vi "rydberg_trigger_snap.vi"() -> ()   [LabVIEW 2013]
uses:
  instrumentvi_Neutral/cameratrigger/related_vi/check_pixelfly_status.vi
  <vilib>/Utility/file.llb/Read From Spreadsheet File (DBL).vi
  <vilib>/Utility/file.llb/Write To Spreadsheet File (DBL).vi
panel:
  in  "Case Constant\n(See Context Help) 2":bool
  in  "Case Constant\n(See Context Help)":bool
  out "iteration#":i32=25
  in  "Turn channels ON/OFF\n(works in real time)":bool[](array[boolean])=[TRUE, TRUE, FALSE, FALSE, FALSE, FALSE, FALSE, FALSE, FALSE, FALSE, FALSE, FALSE, FALSE, FALSE, FALSE, FALSE]
  in  "Save data every nth iteration":dbl=25.0
  out "Analog Input \nVoltage Monitor":T1(graph)={"data[0]"=-0.7588496337314492, "data[1]"=-0.07985869959699164, "data[2]"=0.0, "data[3]"=0.0, "data[4]"=0.0, "data[5]"=0.0, "data[6]"=0.0, "data[7]"=0.0, "data[8]"=0.0, "data[9]"=0.0, "data[10]"=0.0, "data[11]"=0.0, "data[12]"=0.0, "data[13]"=0.0, "data[14]"=0.0, "data[15]"=0.0}
  in  "Tab Control":enum32{"Controls", "Images", "Status"}(tab)=enum."Images"
  in  "Voltage Log File Path":path=path "C:/data/Voltage Log Files/voltagelog011708.txt"
  in  "Monitor voltages?":bool
  in  "Voltage\nMonitor\nControl":u16(ring)=1 caption="Voltage Monitor Control" items=["Off", "Each imaging cycle", "Verdi temp mon"]
  out "DoubleShutter?":bool=TRUE
  in  "File Path for Electronic Background Image":path=path "C:/data/tempfiles/junkeback.dat"
  in  "File Path for Atoms":path=path "C:/data/tempfiles/junkatoms.dat"
  in  "File Path for Background":path=path "C:/data/tempfiles/junkback.dat"
  in  "Timeout (min 100 ms)":u32=1000
  in  "Max Iteration (timeout)":i32=51
  in  "Camera background with no image beam.\nIt will be subtracted before the log is taken":i16 min=0
  in  "Software Bin Size":i32=2
  in  "Software Binning?":bool=TRUE
  in  "Subtract Electronic BG?":bool
  in  "Cut Image?":bool=TRUE
  in  "ROI Parameters":T2={"Col Start"=250, "Col Stop"=550, "Row Start"=1025, "Row stop"=1225} {"Row stop" min=1 max=1280; "Row Start" min=1 max=1280; "Col Stop" min=1 max=1024; "Col Start" min=1 max=1024}
  in  "Coil Current (amps)":dbl=34.0 format="%.2f"
  in  "Natural Linewidth of Transition (in MHz)":dbl=32.0
  in  "Image Beam Detuning (MHz)":dbl format="%.2f"
  in  "Image Beam Wavelength (m)":dbl=4.61e-07
  in  "Number for Scale":dbl=5.0
  in  "Number of Pixels to Smooth":dbl=1.0
  in  "Cut Borders":dbl
  in  "Limit":dbl=5.0
  in  "Sample Interleave":dbl=1.0 min=1.0
  in  "Pixel Size (m)":dbl=6e-06
  in  "Scale Base Level?":bool
  in  "1D Fit On?":bool=TRUE
  in  "2D Fit On?":bool=TRUE
  out "boardid (indicator)":i32
  in  "Gain":i32(ring) items=["Low (X1)", "High (X2)"]
  in  "Exp Time: This sets first image exposure and start of image readout. Make sure you account for this time.":i32=1000 min=1 max=10000
  in  "V Bin":i32(ring) items=["1", "2"]
  in  "H Bin":i32(ring) items=["1", "2"]
  in  "Exp Level":i32=1 min=0 max=255 step=1
  in  "Trigger":bool=TRUE
  in  "Exposure Mode":u16(ring)=1 items=["Asynch shutter", "Double shot", "Video mode", "Auto exposure"]
  out "?":ext format="%.2f"
  in  "?":i32=35
  in  "?":i32=87
  out "PixelFly Status":bool
  out "Atoms - Background at Analysis Size":dbl[][](graph)
  out "image -  bg sum of ROI from back":dbl(graph)=-492168.0
  out "Last 40 numbers":dbl(graph)
  out "Atoms Image":dbl[][](graph)
  out "Atoms - Background":dbl[][](graph)
  out "parameters from \npeak absorption":T3={"alpha"=1.0152277070063695e-13, "peakdensity"=4.819850374584978e+17, "alphadenssigzsqrt2pi"=2.914507, "number"=142895.21998245403} {"number" format="%.3e"; "alphadenssigzsqrt2pi" format="%.3e"; "peakdensity" format="%.3e"; "alpha" format="%.3e"}
  out "Image Size for Analysis":i32[](array[numeric])=[150, 100]
  out "peak OD":dbl format="%#_4g"
  in  "# Images to Sum":i32=1
  in  "Continuous Scan?\n(No Images Saved)":bool=TRUE
  in  "Autoscale\nRoutine On?":bool
  in  "Analyze \nImages?":bool=TRUE
  out "# of Current Image":i32=1
  in  "Camera Function":i32(ring)=2 items=["Camera Initialize", "Acquire", "Shutdown"]
  in  "Stop Continuous Scan?":bool
  out "2D Fit Chi-squared":dbl format="%#_3g"
  out "Num Atoms - OD Integral":dbl format="%#_4g"
  out "Num Atoms - Peak OD":dbl format="%#_4g"
  out "Y 1D Fit Values":T4={"Amplitude"=17.90491094333259, "y0"=0.0006453741239587313, "rmswidthy"=3.333942391455422e-05, "offsety"=-3.142553421752575, "Number Y"=176863.40216585185} {"Number Y" format="%.2e"; "offsety" format="%.2e"; "rmswidthy" format="%.2e"; "y0" format="%.2e"; "Amplitude" format="%.2e"}
  out "X 1D Fit Values":T5={"Amplitude"=24.47847782439825, "x0"=0.0009429207504454069, "rmswidthx"=2.376173376668835e-05, "offsetx"=-2.0737454877905925, "Number X"=172333.71575846447} {"Number X" format="%.2e"; "offsetx" format="%.2e"; "rmswidthx" format="%.2e"; "x0" format="%.2e"; "Amplitude" format="%.2e"}
  out "2-D Fit Parameters":T6
  out "Avg Back":ext=1449.7175567626953 format="%.2e"
  out "Avg Atoms-Back":ext=-7.78399887084961 format="%.2e"
  out "Avg Atoms":ext=1441.9335578918458 format="%.2e"
  out "Opticaldepthimagesingle (ln(atoms)-ln(back))(-1)":dbl[][](graph)
  out "Smoothed OD - Fit OD":dbl[][](graph)
  out "Uncut Image - Doubleshot":dbl[][](graph)
  out "Y density distribution: log(sum_x atoms) -log(sum_x backgnd)":cluster{dbl[], dbl[]}[](graph)=[{[0.0, 1.2e-05, 2.4e-05, 3.6e-05, 4.8e-05, 6e-05, 7.2e-05, 8.400000000000001e-05, 9.6e-05, 0.000108, 0.00012, 0.000132, 0.000144, 0.000156, 0.00016800000000000002, 0.00018, 0.000192, 0.000204, 0.000216, 0.000228, 0.00024, 0.000252, 0.000264, 0.000276, 0.000288, 0.00030000000000000003, 0.000312, 0.000324, 0.00033600000000000004, 0.000348, 0.00036, 0.000372, 0.000384, 0.00039600000000000003, 0.000408, 0.00042, 0.000432, 0.000444, 0.000456, 0.000468, 0.00048, 0.000492, 0.000504, 0.000516, 0.000528, 0.00054, 0.000552, 0.000564, 0.000576, 0.000588, 0.0006000000000000001, 0.000612, 0.000624, 0.0006360000000000001, 0.000648, 0.00066, 0.0006720000000000001, 0.000684, 0.000696, 0.000708, 0.00072, 0.000732, 0.000744, 0.000756, 0.000768, 0.00078, 0.0007920000000000001, 0.000804, 0.000816, 0.0008280000000000001, 0.00084, 0.000852, 0.000864, 0.000876, 0.000888, 0.0009, 0.000912, 0.000924, 0.000936, 0.0009480000000000001, 0.00096, 0.000972, 0.000984, 0.000996, 0.001008, 0.00102, 0.001032, 0.001044, 0.001056, 0.001068, 0.00108, 0.001092, 0.001104, 0.001116, 0.001128, 0.00114, 0.001152, 0.001164, 0.001176, 0.001188], [-3.3686591448665695, -3.3593416907117444, -2.501141797799619, -3.137266718233832, -3.587719306130566, -2.6390745848241295, -3.6966092446853054, -2.6808187998242374, -3.0319112156403207, -2.7363781603955886, -3.363138854673707, -2.731002614818408, -3.3935197594450983, -3.0493035465378853, -3.2941032756557433, -3.092209549305835, -3.0943983454935733, -3.2393686037710268, -2.730035543135955, -3.287849371356515, -2.5686023814239434, -3.1088703551167782, -2.856653458062283, -3.240447915604136, -3.4894394818825276, -2.9961131164766357, -4.104169957056229, -2.8255474959485127, -3.8878748767015168, -3.0775415698653887, -3.7197529539632797, -3.3776657935209187, -3.8047169273982036, -3.4536401406066943, -3.3930728929356064, -3.1293918380520154, -3.433923718918095, -2.8153587940721536, -3.6029531308467995, -2.4989306176071295, -3.483829652183431, -2.9711985693618317, -3.697510544320039, -3.1132099718149675, -3.803881645787669, -3.6495652439025434, -3.6485837854809233, -3.185441611433589, -1.652208255575033, 0.03140941165247568, 4.4569342541294645, 8.56173788023807, 12.377374823114451, 13.49419715605518, 13.361094012986996, 13.08877719779457, 10.635138116352437, 6.592571400876977, 2.8347368854219894, -0.6335944505865427, -2.5137500326873123, -3.043489857024497, -2.68801842384687, -3.0676047259767074, -2.9163649829733913, -3.168337622954141, -2.7690334242099652, -3.322776293644665, -3.119521162448791, -3.04783132514558, -2.619550840819329, -3.2013707187938962, -2.419650797146687, -2.902692626093767, -3.0917951318126597, -2.8856469922691304, -3.523759843666312, -3.0084041621928463, -3.646833134218241, -3.1529925921761333, -3.371597483779624, -3.5211395371050003, -3.153552371623391, -3.4981555573237983, -3.7751962171532796, -2.992402620435996, -3.2399196976318763, -2.831696410884433, -2.7750651929482046, -2.8873123361618127, -2.360377205045097, -2.399998629312904, -2.590436576132106, -2.2120804438281993, -2.5532249988086733, -2.7154620505466482, -2.369902307173561, -3.201516908291751, -2.571788439326383, -2.629373703639885]}, {[0.0, 1.2e-05, 2.4e-05, 3.6e-05, 4.8e-05, 6e-05, 7.2e-05, 8.400000000000001e-05, 9.6e-05, 0.000108, 0.00012, 0.000132, 0.000144, 0.000156, 0.00016800000000000002, 0.00018, 0.000192, 0.000204, 0.000216, 0.000228, 0.00024, 0.000252, 0.000264, 0.000276, 0.000288, 0.00030000000000000003, 0.000312, 0.000324, 0.00033600000000000004, 0.000348, 0.00036, 0.000372, 0.000384, 0.00039600000000000003, 0.000408, 0.00042, 0.000432, 0.000444, 0.000456, 0.000468, 0.00048, 0.000492, 0.000504, 0.000516, 0.000528, 0.00054, 0.000552, 0.000564, 0.000576, 0.000588, 0.0006000000000000001, 0.000612, 0.000624, 0.0006360000000000001, 0.000648, 0.00066, 0.0006720000000000001, 0.000684, 0.000696, 0.000708, 0.00072, 0.000732, 0.000744, 0.000756, 0.000768, 0.00078, 0.0007920000000000001, 0.000804, 0.000816, 0.0008280000000000001, 0.00084, 0.000852, 0.000864, 0.000876, 0.000888, 0.0009, 0.000912, 0.000924, 0.000936, 0.0009480000000000001, 0.00096, 0.000972, 0.000984, 0.000996, 0.001008, 0.00102, 0.001032, 0.001044, 0.001056, 0.001068, 0.00108, 0.001092, 0.001104, 0.001116, 0.001128, 0.00114, 0.001152, 0.001164, 0.001176, 0.001188], [-3.142553421752575, -3.142553421752575, -3.142553421752575, -3.142553421752575, -3.142553421752575, -3.142553421752575, -3.142553421752575, -3.142553421752575, -3.142553421752575, -3.142553421752575, -3.142553421752575, -3.142553421752575, -3.142553421752575, -3.142553421752575, -3.142553421752575, -3.142553421752575, -3.142553421752575, -3.142553421752575, -3.142553421752575, -3.142553421752575, -3.142553421752575, -3.142553421752575, -3.142553421752575, -3.142553421752575, -3.142553421752575, -3.142553421752575, -3.142553421752575, -3.142553421752575, -3.142553421752575, -3.142553421752575, -3.142553421752573, -3.14255342175253, -3.1425534217517685, -3.1425534217398705, -3.1425534215767574, -3.142553419615115, -3.142553398924452, -3.142553207572838, -3.1425516564361646, -3.1425406396371858, -3.1424721164431455, -3.1420990921048606, -3.1403231424865408, -3.1329354518498045, -3.106116340729864, -3.021287229549591, -2.788007984145684, -2.231927393950265, -1.0878733189191243, 0.9301648516208109, 3.9493125759985808, 7.706020947338827, 11.43621434642004, 14.068401345797076, 14.706907582526853, 13.11971957540532, 9.873322089660576, 6.009141262246697, 2.510273096557114, -0.0751860764137236, -1.680369782741332, -2.530239620690055, -2.917294410160682, -3.0697542735255157, -3.1218850426129303, -3.137398494519852, -3.1414239518658547, -3.1423360201347044, -3.1425166607891493, -3.1425479610692, -3.1425527091570276, -3.142553340061387, -3.1425534135255404, -3.142553421024716, -3.1425534216960047, -3.1425534217487128, -3.142553421752343, -3.142553421752563, -3.1425534217525746, -3.142553421752575, -3.142553421752575, -3.142553421752575, -3.142553421752575, -3.142553421752575, -3.142553421752575, -3.142553421752575, -3.142553421752575, -3.142553421752575, -3.142553421752575, -3.142553421752575, -3.142553421752575, -3.142553421752575, -3.142553421752575, -3.142553421752575, -3.142553421752575, -3.142553421752575, -3.142553421752575, -3.142553421752575, -3.142553421752575, -3.142553421752575]}]
  out "Intensity v/s X":cluster{dbl[], dbl[]}[](graph)=[{[0.0, 1.2e-05, 2.4e-05, 3.6e-05, 4.8e-05, 6e-05, 7.2e-05, 8.400000000000001e-05, 9.6e-05, 0.000108, 0.00012, 0.000132, 0.000144, 0.000156, 0.00016800000000000002, 0.00018, 0.000192, 0.000204, 0.000216, 0.000228, 0.00024, 0.000252, 0.000264, 0.000276, 0.000288, 0.00030000000000000003, 0.000312, 0.000324, 0.00033600000000000004, 0.000348, 0.00036, 0.000372, 0.000384, 0.00039600000000000003, 0.000408, 0.00042, 0.000432, 0.000444, 0.000456, 0.000468, 0.00048, 0.000492, 0.000504, 0.000516, 0.000528, 0.00054, 0.000552, 0.000564, 0.000576, 0.000588, 0.0006000000000000001, 0.000612, 0.000624, 0.0006360000000000001, 0.000648, 0.00066, 0.0006720000000000001, 0.000684, 0.000696, 0.000708, 0.00072, 0.000732, 0.000744, 0.000756, 0.000768, 0.00078, 0.0007920000000000001, 0.000804, 0.000816, 0.0008280000000000001, 0.00084, 0.000852, 0.000864, 0.000876, 0.000888, 0.0009, 0.000912, 0.000924, 0.000936, 0.0009480000000000001, 0.00096, 0.000972, 0.000984, 0.000996, 0.001008, 0.00102, 0.001032, 0.001044, 0.001056, 0.001068, 0.00108, 0.001092, 0.001104, 0.001116, 0.001128, 0.00114, 0.001152, 0.001164, 0.001176, 0.001188, 0.0012000000000000001, 0.001212, 0.001224, 0.0012360000000000001, 0.001248, 0.00126, 0.0012720000000000001, 0.001284, 0.001296, 0.0013080000000000001, 0.00132, 0.001332, 0.0013440000000000001, 0.001356, 0.001368, 0.00138, 0.001392, 0.001404, 0.001416, 0.001428, 0.00144, 0.001452, 0.001464, 0.001476, 0.001488, 0.0015, 0.001512, 0.001524, 0.001536, 0.0015480000000000001, 0.00156, 0.001572, 0.0015840000000000001, 0.001596, 0.001608, 0.0016200000000000001, 0.001632, 0.001644, 0.0016560000000000001, 0.001668, 0.00168, 0.0016920000000000001, 0.001704, 0.001716, 0.001728, 0.00174, 0.001752, 0.001764, 0.001776, 0.001788], [-2.8183440721355737, -2.401522563761773, -2.5237601060707675, -2.500570399573121, -2.506086929574394, -2.3798757992705077, -2.491986345524083, -2.488259685244998, -2.5954764602082605, -2.6088044268195745, -2.565883062250009, -2.640123527845276, -2.5258645679890606, -2.542319425147525, -2.3663141562295777, -2.491158449081013, -2.4827761290987382, -2.5697565230360624, -2.675555471134544, -2.4526500510070264, -2.587401679302161, -2.7170704998887913, -2.5610989943488676, -2.5911334487145723, -2.5002374964478804, -2.4884694389456854, -2.5394904176372393, -2.5500867554972046, -2.378216817131488, -2.5395407567208395, -2.046418844121149, -2.1733857420010736, -2.669858427788313, -2.2304504062857404, -2.586975439308276, -2.4213636413369386, -2.3929041134997533, -2.488418399790703, -2.2930625821045396, -2.6069475160815045, -2.511643300766991, -2.273400532704045, -2.2899489155247466, -2.528198542008795, -2.357612131615724, -2.3432177912642373, -2.3168511287027513, -2.420032372065748, -2.395414080287992, -2.3757390661600084, -2.4716707833126748, -2.2185297028257764, -2.2814791274250865, -2.118623996360043, -2.0182357551965424, -2.432618062946176, -2.230506420081042, -2.146155705062938, -2.3472190640306962, -2.3712543536693147, -2.1875881775472408, -2.1952908358917966, -2.053287952368919, -1.8502300747721847, -1.9848473505809352, -1.9942680470508094, -2.0174521250165753, -2.0969782433525097, -1.8219170436304921, -1.6672326334789886, -1.4869217102946095, -0.9996339197143698, -0.8098748137616667, -0.35967428953222225, -0.650012388682967, 1.7919178156766975, 7.743635801250548, 16.428591835436464, 22.663725551287143, 20.240706904645776, 16.936256193013378, 9.701135845766885, 4.174916332451744, -0.2899352730639748, -1.661331740025389, -1.5080821335172914, -1.9026215949503467, -2.049002401491748, -1.9706402437938095, -2.0311585837459916, -2.077597516112178, -1.930667645093763, -2.1086022731634557, -1.7650030212055299, -1.917311464733416, -1.8111299981898128, -2.075459160990931, -2.2079166808241553, -1.8235763980834463, -1.898222513860219, -1.9621602868612626, -2.0017564868267073, -1.7095965014406147, -2.0323342222595784, -1.6211606697328307, -1.839833902685882, -1.9658503587635323, -1.9776012347161895, -1.887885369120113, -1.9468724100556756, -1.6351243930344026, -1.6613815392586275, -1.6219275265368651, -1.7589024364108354, -1.6045421848466503, -1.8391976965150434, -1.6203149700231734, -1.7969550536250836, -1.5575704192364128, -1.8258635266791998, -1.9097093493073771, -1.8343058761104203, -1.660627277068329, -1.945166122309729, -1.5463727138680952, -1.569489672727741, -1.6225878206881816, -1.7324496472705277, -1.631544148883222, -1.8227215123275755, -1.8797703918872912, -1.8647363562896544, -1.576905869043685, -1.970412155507347, -2.0096411488008243, -1.7813961287674829, -1.8489792019571496, -1.7513334844093151, -1.6826445124467, -1.8905109948545942, -1.7110939804845202, -1.7394070082149256, -1.599355827269278, -1.686777376633131, -1.4884369858077662, -1.653664890583741, -1.8092625318996625, -1.4833808568982931, -1.6619157448002397, -1.371210367738854]}, {[0.0, 1.2e-05, 2.4e-05, 3.6e-05, 4.8e-05, 6e-05, 7.2e-05, 8.400000000000001e-05, 9.6e-05, 0.000108, 0.00012, 0.000132, 0.000144, 0.000156, 0.00016800000000000002, 0.00018, 0.000192, 0.000204, 0.000216, 0.000228, 0.00024, 0.000252, 0.000264, 0.000276, 0.000288, 0.00030000000000000003, 0.000312, 0.000324, 0.00033600000000000004, 0.000348, 0.00036, 0.000372, 0.000384, 0.00039600000000000003, 0.000408, 0.00042, 0.000432, 0.000444, 0.000456, 0.000468, 0.00048, 0.000492, 0.000504, 0.000516, 0.000528, 0.00054, 0.000552, 0.000564, 0.000576, 0.000588, 0.0006000000000000001, 0.000612, 0.000624, 0.0006360000000000001, 0.000648, 0.00066, 0.0006720000000000001, 0.000684, 0.000696, 0.000708, 0.00072, 0.000732, 0.000744, 0.000756, 0.000768, 0.00078, 0.0007920000000000001, 0.000804, 0.000816, 0.0008280000000000001, 0.00084, 0.000852, 0.000864, 0.000876, 0.000888, 0.0009, 0.000912, 0.000924, 0.000936, 0.0009480000000000001, 0.00096, 0.000972, 0.000984, 0.000996, 0.001008, 0.00102, 0.001032, 0.001044, 0.001056, 0.001068, 0.00108, 0.001092, 0.001104, 0.001116, 0.001128, 0.00114, 0.001152, 0.001164, 0.001176, 0.001188, 0.0012000000000000001, 0.001212, 0.001224, 0.0012360000000000001, 0.001248, 0.00126, 0.0012720000000000001, 0.001284, 0.001296, 0.0013080000000000001, 0.00132, 0.001332, 0.0013440000000000001, 0.001356, 0.001368, 0.00138, 0.001392, 0.001404, 0.001416, 0.001428, 0.00144, 0.001452, 0.001464, 0.001476, 0.001488, 0.0015, 0.001512, 0.001524, 0.001536, 0.0015480000000000001, 0.00156, 0.001572, 0.0015840000000000001, 0.001596, 0.001608, 0.0016200000000000001, 0.001632, 0.001644, 0.0016560000000000001, 0.001668, 0.00168, 0.0016920000000000001, 0.001704, 0.001716, 0.001728, 0.00174, 0.001752, 0.001764, 0.001776, 0.001788], [-2.0737454877905925, -2.0737454877905925, -2.0737454877905925, -2.0737454877905925, -2.0737454877905925, -2.0737454877905925, -2.0737454877905925, -2.0737454877905925, -2.0737454877905925, -2.0737454877905925, -2.0737454877905925, -2.0737454877905925, -2.0737454877905925, -2.0737454877905925, -2.0737454877905925, -2.0737454877905925, -2.0737454877905925, -2.0737454877905925, -2.0737454877905925, -2.0737454877905925, -2.0737454877905925, -2.0737454877905925, -2.0737454877905925, -2.0737454877905925, -2.0737454877905925, -2.0737454877905925, -2.0737454877905925, -2.0737454877905925, -2.0737454877905925, -2.0737454877905925, -2.0737454877905925, -2.0737454877905925, -2.0737454877905925, -2.0737454877905925, -2.0737454877905925, -2.0737454877905925, -2.0737454877905925, -2.0737454877905925, -2.0737454877905925, -2.0737454877905925, -2.0737454877905925, -2.0737454877905925, -2.0737454877905925, -2.0737454877905925, -2.0737454877905925, -2.0737454877905925, -2.0737454877905925, -2.0737454877905925, -2.0737454877905925, -2.0737454877905925, -2.0737454877905925, -2.0737454877905925, -2.0737454877905925, -2.0737454877905925, -2.0737454877905925, -2.0737454877905925, -2.0737454877905925, -2.0737454877905925, -2.0737454877905925, -2.0737454877905925, -2.0737454877905925, -2.0737454877905925, -2.073745487790578, -2.073745487789698, -2.073745487748773, -2.0737454862751323, -2.073745445235809, -2.0737445618346193, -2.073729875366191, -2.073541507399717, -2.0716803713160936, -2.0575446026371003, -1.9752602822028478, -1.6098273966897678, -0.3803839855887031, 2.715820000636734, 8.423627049166667, 15.754276644617699, 21.388186935825832, 21.85183342897553, 16.8322343699678, 9.50266684232387, 3.41896670995723, -0.05427383695049559, -1.4984026137046382, -1.9467308492977926, -2.052017531704562, -2.0708652918518737, -2.0734496434587752, -2.0737219404138356, -2.0737440354787706, -2.073745418381675, -2.073745485220145, -2.0737454877168293, -2.073745487788952, -2.073745487790564, -2.073745487790592, -2.0737454877905925, -2.0737454877905925, -2.0737454877905925, -2.0737454877905925, -2.0737454877905925, -2.0737454877905925, -2.0737454877905925, -2.0737454877905925, -2.0737454877905925, -2.0737454877905925, -2.0737454877905925, -2.0737454877905925, -2.0737454877905925, -2.0737454877905925, -2.0737454877905925, -2.0737454877905925, -2.0737454877905925, -2.0737454877905925, -2.0737454877905925, -2.0737454877905925, -2.0737454877905925, -2.0737454877905925, -2.0737454877905925, -2.0737454877905925, -2.0737454877905925, -2.0737454877905925, -2.0737454877905925, -2.0737454877905925, -2.0737454877905925, -2.0737454877905925, -2.0737454877905925, -2.0737454877905925, -2.0737454877905925, -2.0737454877905925, -2.0737454877905925, -2.0737454877905925, -2.0737454877905925, -2.0737454877905925, -2.0737454877905925, -2.0737454877905925, -2.0737454877905925, -2.0737454877905925, -2.0737454877905925, -2.0737454877905925, -2.0737454877905925, -2.0737454877905925, -2.0737454877905925, -2.0737454877905925, -2.0737454877905925, -2.0737454877905925, -2.0737454877905925, -2.0737454877905925, -2.0737454877905925]}] caption="X Density Distribution: log(sum_y atoms) -log(sum_y backgnd)"
  out "Background Image":dbl[][](graph)
  out "Strip Chart\nerror out":errorcluster
  in  "Strip Chart\nerror in":errorcluster
  out "Strip chart counter":dbl
  out "initialized array":u8[][](array[numeric])
  in  "error in":errorcluster
  out "error out":errorcluster={"status"=TRUE, "code"=-131, "source"="Remove buffer from list.vi: Picture buffer already in use"} caption="Camera Error Out 1"
  out "error out 2":errorcluster={"status"=FALSE, "code"=0, "source"="Start camera.vi: No error - function call successful"} caption="Camera Error Out 2"
  out "Camera Error Out 3":errorcluster={"status"=FALSE, "code"=0, "source"="Get buffer status.vi: No error - function call successful"}
  out "V bin 2":i32(ring) items=["1", "2"]
  out "H bin 2":i32(ring) items=["1", "2"]
  out "Buffer number":i32=1
  out "Size":i32=5242880
  out "Buffer address":i32=241958912
  out "Camera Board Parameters":T7={"Type"=65, "Number"=1, "Initialized"=TRUE, "Running"=TRUE, "Lost head"=FALSE, "CCD X size"=1280, "CCD Y size"=1024, "Mode"=32, "Exposure time"=1000, "Exposure level"=1, "Horizontal bin"=0, "Vertical bin"=0, "Reg W"=FALSE, "Gain"=0, "Pixel depth"=12, "Bit Shift"=0, "Offset"=0, "Last exposure"=1000, "Double "=TRUE, "Light meter"=FALSE, "Color"=FALSE, "Open count"=2295301936, "Active buffer"=TRUE, "Next Buffer"=TRUE} {"Vertical bin" items=["1", "2"]; "Horizontal bin" items=["1", "2"]}
  out "Camera Buffer status":T8={"Write"=FALSE, "Write done"=TRUE, "Queued"=FALSE, "Cancelled"=FALSE, "Select"=FALSE, "Select done"=FALSE, "Burst"=FALSE, "Size"=FALSE, "Event"=FALSE, "Timeout"=FALSE, "Open"=0, "Map"=4372, "Exposure"=[1000], "Offset"=[0], "Size"=[5242880], "Transfer"=[0], "Total Size"=392691712}
  in  "offset":i32
  out "Output ClusterY\n(arb fit)":T9={"amplitudey"=0.008995711509471623, "temperaturey"=0.002709094402736608, "alphay"=0.0011778671316246122, "offsety"=-0.0002344292151486787, "numbery"=771798750.645837, "peakdensityy"=4696134676573208.0, "centery"=0.004923587672892697} {"centery" format="%.2e"; "peakdensityy" format="%.2e"; "numbery" format="%.2e"; "offsety" format="%.2e"; "alphay" format="%.2e"; "temperaturey" format="%.2e"; "amplitudey" format="%.2e"}
  out "Output Cluster X\n(arb fit)":T10={"amplitudex"=0.0047697219685124154, "temperaturex"=0.0023439442598952344, "alphax"=0.0010191061999544498, "offsetx"=8.440276213188199e-05, "numberx"=708132868.1536969, "peakdensityx"=6652452808873044.0, "centerx"=0.0037182148271134325} {"centerx" format="%.2e"; "peakdensityx" format="%.2e"; "numberx" format="%.2e"; "offsetx" format="%.2e"; "alphax" format="%.2e"; "temperaturex" format="%.2e"; "amplitudex" format="%.2e"}
  out "Y side(by arbfit)":cluster{cluster{dbl, dbl}[]}[](graph)=[{[{0.0, -9.666143798828125e-05}, {4.63e-05, 4.321251220703125e-05}, {9.26e-05, -0.00016961046142578126}, {0.00013890000000000002, -0.0001606823974609375}, {0.0001852, -3.920782470703125e-05}, {0.0002315, -0.000111915087890625}, {0.00027780000000000003, -0.00018772257080078126}, {0.0003241, -0.00014607723388671877}, {0.0003704, 3.730218505859375e-05}, {0.0004167, -0.000120493310546875}, {0.000463, -2.0831201171875e-05}, {0.0005093, 8.1265576171875e-05}, {0.0005556000000000001, -4.6981127929687503e-05}, {0.0006019, 2.730753173828125e-05}, {0.0006482, 0.0001042299560546875}, {0.0006945, 8.897061767578125e-05}, {0.0007408, -0.0001128991943359375}, {0.0007871, -3.39658935546875e-05}, {0.0008334, 0.00021708648681640627}, {0.0008797, 1.521951904296875e-05}, {0.000926, -8.81429443359375e-05}, {0.0009723, 0.00017849017333984376}, {0.0010186, 0.00016118013916015624}, {0.0010649, 4.3130029296875e-05}, {0.0011112000000000001, 0.000101584814453125}, {0.0011575000000000001, 0.0001667121826171875}, {0.0012038, 0.0001330364013671875}, {0.0012501, 1.435771484375e-05}, {0.0012964, 0.00013017509765625}, {0.0013427, 0.0001979874267578125}, {0.001389, 0.0001995517578125}, {0.0014353, 5.386134033203125e-05}, {0.0014816, 0.00013825557861328125}, {0.0015279, 0.00037487060546875003}, {0.0015742, 0.0001915253173828125}, {0.0016205, 0.000173282373046875}, {0.0016668, 0.00030387272949218753}, {0.0017131, 0.0005522344604492188}, {0.0017594, 0.0003743757080078125}, {0.0018057, 0.000244183544921875}, {0.001852, 0.0004390764404296875}, {0.0018983000000000001, 0.0004536360961914063}, {0.0019446, 0.00044938680419921874}, {0.0019909, 0.00031516435546875}, {0.0020372, 0.0003973002685546875}, {0.0020835, 0.000558414990234375}, {0.0021298, 0.0005315966674804687}, {0.0021761, 0.00047105989990234374}, {0.0022224000000000002, 0.0006024039794921875}, {0.0022687000000000002, 0.0006190456176757812}, {0.0023150000000000002, 0.0006605089233398438}, {0.0023613, 0.0006151063476562501}, {0.0024076, 0.0007049785888671875}, {0.0024539, 0.0008554387939453125}, {0.0025002, 0.000755099755859375}, {0.0025465, 0.0008008635498046875}, {0.0025928, 0.0007846542358398437}, {0.0026391, 0.00092633427734375}, {0.0026854, 0.0009349409423828125}, {0.0027317, 0.0009390679321289063}, {0.002778, 0.0009715178466796875}, {0.0028243, 0.0009944736938476563}, {0.0028706, 0.001180484033203125}, {0.0029169, 0.0010933195068359375}, {0.0029632, 0.0010906231689453126}, {0.0030095, 0.0010906317016601563}, {0.0030558, 0.0013240981567382813}, {0.0031021, 0.0014536930297851564}, {0.0031484, 0.001447785546875}, {0.0031947, 0.0013987793212890626}, {0.003241, 0.0015179443725585938}, {0.0032873, 0.0015591374755859375}, {0.0033336, 0.0016731800537109376}, {0.0033799, 0.0016079417602539064}, {0.0034262, 0.0015991075561523438}, {0.0034725, 0.0018513971801757813}, {0.0035188, 0.0018405805419921875}, {0.0035651, 0.0018605926025390626}, {0.0036114, 0.001904240283203125}, {0.0036577, 0.0018782012817382813}, {0.003704, 0.0019519751342773437}, {0.0037503000000000002, 0.0020929782470703127}, {0.0037966000000000002, 0.002198195153808594}, {0.0038429000000000002, 0.0021514216552734377}, {0.0038892, 0.0020961069091796876}, {0.0039355, 0.002265489831542969}, {0.0039818, 0.0023468663330078127}, {0.0040281, 0.002427193310546875}, {0.0040744, 0.0024689637939453125}, {0.0041207, 0.0024438804565429686}, {0.004167, 0.0024601580322265626}, {0.0042133, 0.002636688525390625}, {0.0042596, 0.002699147998046875}, {0.0043059, 0.002643045397949219}, {0.0043522, 0.0026505143676757814}, {0.0043985, 0.0026222966796875}, {0.0044448000000000005, 0.0027097114990234377}, {0.0044911000000000005, 0.0027219531005859376}, {0.0045374000000000005, 0.0027993960205078125}, {0.0045837000000000004, 0.002850597998046875}, {0.0046300000000000004, 0.0028023995361328127}, {0.0046763, 0.0027945295288085937}, {0.0047226, 0.0029437581787109374}, {0.0047689, 0.0029110010864257813}, {0.0048152, 0.0030008591064453125}, {0.0048615, 0.002974151708984375}, {0.0049078, 0.002937995751953125}, {0.0049541, 0.0029096813598632814}, {0.0050004, 0.0029673767333984378}, {0.0050467, 0.003066478527832031}, {0.005093, 0.00306333564453125}, {0.0051393, 0.003041998168945313}, {0.0051856, 0.0028867596435546874}, {0.0052319, 0.0027757006713867187}, {0.0052782, 0.0028882158935546877}, {0.0053245, 0.0029104151733398437}, {0.0053708, 0.0027892534667968752}, {0.0054171, 0.0027464476806640624}, {0.0054634, 0.002764500061035156}, {0.0055097, 0.0026023215942382813}, {0.005556, 0.0025186128173828124}, {0.0056023, 0.002569339807128906}, {0.0056486, 0.0024484426147460938}, {0.0056949, 0.0024748428344726564}, {0.0057412, 0.002454739758300781}, {0.0057875, 0.0023008465576171877}, {0.0058338, 0.0023179062988281252}, {0.0058801, 0.00228233056640625}, {0.0059264, 0.0022157355712890624}, {0.0059727, 0.0020830091918945313}, {0.006019, 0.002083563818359375}, {0.0060653, 0.0020847953735351563}, {0.0061116, 0.002062195056152344}, {0.0061579, 0.0019736823608398437}, {0.0062042, 0.0018520598876953125}, {0.0062505, 0.0018948542968750001}, {0.0062968, 0.0017422921997070314}, {0.0063431, 0.0016028676391601562}, {0.0063894, 0.0016803645996093751}, {0.0064357, 0.0015904127197265625}, {0.006482, 0.0015004665283203126}, {0.0065283, 0.001450151953125}, {0.0065746, 0.0014172981567382812}, {0.0066209, 0.001336484814453125}, {0.0066672, 0.00135934111328125}, {0.0067135, 0.001208789892578125}, {0.0067598, 0.0012902744750976562}, {0.0068061, 0.0011487451782226563}, {0.0068524, 0.001103211767578125}, {0.0068987, 0.0011628611328125}, {0.006945, 0.0011180217163085937}, {0.0069913, 0.00104233369140625}, {0.0070376, 0.001006120849609375}, {0.0070839, 0.0009368323608398438}, {0.0071302, 0.0008879626586914063}, {0.0071765, 0.0008855393676757813}, {0.0072228, 0.0007939548950195313}, {0.0072691, 0.0007488623413085938}, {0.0073154, 0.0007369250732421875}, {0.0073617, 0.0007228916015625}, {0.007408, 0.0006716412719726563}, {0.0074543000000000005, 0.0006353601684570313}, {0.0075006000000000005, 0.0006309515991210938}, {0.0075469000000000005, 0.0005209734375}, {0.0075932000000000005, 0.0005503174438476563}, {0.0076395000000000005, 0.0005640096069335937}, {0.0076858000000000004, 0.0005803668212890625}, {0.0077321, 0.00046943583984375}, {0.0077784, 0.0004919138549804688}, {0.0078247, 0.0004567334716796875}, {0.007871, 0.0004032162841796875}, {0.0079173, 0.0003256823486328125}, {0.0079636, 0.00034895675048828126}, {0.0080099, 0.0002296722412109375}, {0.0080562, 0.00032278122558593753}, {0.0081025, 0.00024264196777343752}, {0.0081488, 0.0002704131103515625}, {0.0081951, 0.0002514306640625}, {0.0082414, 0.00023038614501953125}, {0.0082877, 0.00023180257568359376}]}, {[{0.0, -0.00010865906187833456}, {4.63e-05, -0.00010248175881259633}, {9.26e-05, -9.60946713894237e-05}, {0.00013890000000000002, -8.949093944564066e-05}, {0.0001852, -8.266349606890666e-05}, {0.0002315, -7.560506264006202e-05}, {0.00027780000000000003, -6.830814386093194e-05}, {0.0003241, -6.076502277862111e-05}, {0.0003704, -5.296775581859711e-05}, {0.0004167, -4.4908167840241404e-05}, {0.000463, -3.657784723005229e-05}, {0.0005093, -2.7968141049325046e-05}, {0.0005556000000000001, -1.9070150254923014e-05}, {0.0006019, -9.874725013701312e-06}, {0.0006482, -3.724601332668094e-07}, {0.0006945, 9.446309365930862e-06}, {0.0007408, 1.9591512509667256e-05}, {0.0007871, 3.0073346429921213e-05}, {0.0008334, 4.090228019253389e-05}, {0.0008797, 5.2089058356076504e-05}, {0.000926, 6.364470422192584e-05}, {0.0009723, 7.558052273170855e-05}, {0.0010186, 8.79081029641e-05}, {0.0010649, 0.00010063932017842472}, {0.0011112000000000001, 0.00011378633734756733}, {0.0011575000000000001, 0.0001273616061173385}, {0.0012038, 0.00014137786712360722}, {0.0012501, 0.00015584814959217083}, {0.0012964, 0.00017078577013944924}, {0.0013427, 0.0001862043306846068}, {0.001389, 0.00020211771537558232}, {0.0014353, 0.00021854008642268471}, {0.0014816, 0.00023548587872383942}, {0.0015279, 0.00025296979315517985}, {0.0015742, 0.00027100678838941274}, {0.0016205, 0.00028961207109216836}, {0.0016668, 0.00030880108433330974}, {0.0017131, 0.00032858949403583845}, {0.0017594, 0.0003489931732695157}, {0.0018057, 0.00037002818417953464}, {0.001852, 0.0003917107573224413}, {0.0018983000000000001, 0.00041405726816191505}, {0.0019446, 0.00043708421045589795}, {0.0019909, 0.00046080816624380496}, {0.0020372, 0.00048524577211806353}, {0.0020835, 0.0005104136814379354}, {0.0021298, 0.0005363285221153792}, {0.0021761, 0.0005630068495725409}, {0.0022224000000000002, 0.0005904650944382619}, {0.0022687000000000002, 0.0006187195045167119}, {0.0023150000000000002, 0.0006477860805248956}, {0.0023613, 0.0006776805050573274}, {0.0024076, 0.0007084180641957342}, {0.0024539, 0.000740013561139293}, {0.0025002, 0.0007724812211868801}, {0.0025465, 0.0008058345873573525}, {0.0025928, 0.0008400864058874109}, {0.0026391, 0.0008752485007996484}, {0.0026854, 0.0009113316366866587}, {0.0027317, 0.0009483453688115168}, {0.002778, 0.0009862978795816956}, {0.0028243, 0.0010251958004140647}, {0.0028706, 0.0010650440179748686}, {0.0029169, 0.0011058454637528246}, {0.0029632, 0.0011476008859085435}, {0.0030095, 0.0011903086023428125}, {0.0030558, 0.0012339642339440908}, {0.0031021, 0.0012785604170168652}, {0.0031484, 0.0013240864939633146}, {0.0031947, 0.0013705281813981287}, {0.003241, 0.0014178672150286608}, {0.0032873, 0.001466080970839556}, {0.0033336, 0.0015151420623937199}, {0.0033799, 0.0015650179144126902}, {0.0034262, 0.0016156703132432844}, {0.0034725, 0.001667054935369524}, {0.0035188, 0.0017191208558060519}, {0.0035651, 0.0017718100390292427}, {0.0036114, 0.0018250568160826273}, {0.0036577, 0.0018787873526509141}, {0.003704, 0.0019329191142461635}, {0.0037503000000000002, 0.00198736033620042}, {0.0037966000000000002, 0.0020420095079141044}, {0.0038429000000000002, 0.0020967548827606724}, {0.0038892, 0.0021514740271722454}, {0.0039355, 0.0022060334246843507}, {0.0039818, 0.0022602881530293956}, {0.0040281, 0.0023140816546324302}, {0.0040744, 0.002367245622930107}, 